vi "AeroQuadConfigurator.vi"() -> ()   [LabVIEW 2009]
uses:
  <vilib>/Utility/config.llb/Config Data RefNum.ctl
  <vilib>/Utility/config.llb/Read Key (Double).vi
  <vilib>/Utility/config.llb/Read Key (String).vi
  <vilib>/Utility/config.llb/Write Key (String).vi
  <vilib>/Utility/config.llb/Write Key (U32).vi
  <vilib>/Instr/_visa.llb/VISA Configure Serial Port (Instr).vi
  Instance           2 29Saved   MikroQuadConfigurator .vi
  <vilib>/Utility/error.llb/DialogType.ctl
  <vilib>/Utility/config.llb/NI_LVConfig.lvlib
  <vilib>/ptbypt/NI_PtbyPt.lvlib
panel:
  in  "ConfigGUI":T1(tab)
  in  "Communication Port":refnum<visa-resource-name>
  in  "Timeout (sec)":u32=4
  in  "Connect":bool
  in  "Disconnect":bool
  in  "UpdateAcro":bool
  in  "ProportionalPitch":dbl caption="Proportional" format="%.2f"
  in  "IntegralPitch":dbl caption="Integral" format="%.2f"
  in  "DerivativePitch":dbl caption="Derivative" format="%.2f"
  in  "Proportional Roll":dbl caption="Proportional" format="%.2f"
  in  "Integral Roll":dbl caption="Integral" format="%.2f"
  in  "Derivative Roll":dbl caption="Derivative" format="%.2f"
  in  "Windup Guard":dbl format="%.2f"
  in  "UpdateStable":bool
  in  "ProportionalRollLevel":dbl caption="Proportional" format="%.2f"
  in  "IntegralRollLevel":dbl caption="Integral" format="%.2f"
  in  "DerivativeRollLevel":dbl caption="Derivative" format="%.2f"
  in  "ProportionalPitchLevel":dbl caption="Proportional" format="%.2f"
  in  "IntegralPitchLevel":dbl caption="Integral" format="%.2f"
  in  "DerivativePitchLevel":dbl caption="Derivative" format="%.2f"
  in  "Level Limit":u16
  in  "Level Off":u16=1 min=1 step=1
  in  "ProportionalHeading":dbl caption="Proportional" format="%.2f"
  in  "IntegralHeading":dbl caption="Integral" format="%.2f"
  in  "DerivativeHeading":dbl caption="Derivative" format="%.2f"
  in  "ProportionalYaw":dbl caption="Proportional" format="%.2f"
  in  "IntegralYaw":dbl caption="Integral" format="%.2f"
  in  "DerivativeYaw":dbl caption="Derivative" format="%.2f"
  in  "UpdateYaw":bool
  in  "Gyro Smooth Factor":dbl=0.01 min=0.01 max=1.0 step=0.01 format="%.2f"
  in  "Acc Smooth Factor":dbl=0.01 min=0.01 max=1.0 step=0.01 format="%.2f"
  in  "Complementary Filter":dbl format="%.2f"
  in  "UpdateSensors":bool
  in  "CalibrateGyros":bool
  in  "CalibrateAccels":bool
  in  "Throttle Smoothing":dbl=0.01 min=0.01 max=1.0 step=0.01 format="%.2f"
  in  "Mode  Smoothing":dbl=0.01 min=0.01 max=1.0 step=0.01 format="%.2f"
  in  "Aux  Smoothing":dbl=0.01 min=0.01 max=1.0 step=0.01 format="%.2f"
  in  "Roll Smoothing":dbl=0.01 min=0.01 max=1.0 step=0.01 format="%.2f"
  in  "Pitch Smoothing":dbl=0.01 min=0.01 max=1.0 step=0.01 format="%.2f"
  in  "Yaw  Smoothing":dbl=0.01 min=0.01 max=1.0 step=0.01 format="%.2f"
  in  "UpdateXmit":bool
  in  "Transmitter Factor":dbl=0.01 min=0.01 max=1.0 step=0.01 format="%.2f"
  in  "CalibrateTransmitter":bool
  in  "DefaultTransmitterValue":bool
  in  "Transmitter Instructions 2":string="Before starting the transmitter calibration, set the transmitter to it's default settings.\n\nIt can be in Airplane or Helicopter mode.\n\nVerify that:\n- ESC's and motors are\n  disconnected from power! \n- Trims and subtrims are zero\n- End Point Adjustment (EPA) \n  are 100%"
  in  "Test Comments":string
  in  "SaveFlightData":bool
  in  "ViewFlightData":bool
  in  "InitializeEEPROM":bool
  in  "CalibrateTransmitterFront":bool
  in  "CalibrateESCs":bool
  in  "Minimum Test Throttle":dbl=1050.0 min=1000.0 max=1200.0
  in  "EEPROM Instructions":string="The first step to setting up your AeroQuad is to initialize the user configurable EEPROM with default values. \n\nSelect the \"Initialize EEPROM\" button to set the EEPROM to default values."
  in  "Transmitter Instructions":string="The next step is to calibrate your transmitter. Before starting the calibration, set the\ntransmitter to it's default settings.\n\nIt can be in Airplane or Helicopter mode.\n\nVerify that:\n- ESC's and motors are\n  disconnected from power! \n- Trims and subtrims are zero\n- End Point Adjustment (EPA) \n  are 100%"
  in  "ESC Instructions":string="Before your first flight, perform an ESC throttle calibration per the manufacturer's instructions.  This cal procedure is implemented specifically for the Turnigy line of ESC's.\n\nThe flight control board will need to be powered separately from the ESC's motors.  Use the USB cable to power the flight control board, and a battery to power the ESC's/motors.\n\nInsure that there is no power applied to the ESC's and motors before the start of calibration."
  in  "PerformPreFlightCheckout":bool
  in  "GUI":T2(tab)
  out "Yaw":i16(knob) scale=-200.0..200.0
  out "Pitch":i16(knob) scale=-200.0..200.0
  out "Rear Motor":i16(slide) scale=1000.0..2000.0
  out "Front Motor":i16(slide) scale=1000.0..2000.0
  out "Left Motor":i16(slide) scale=1000.0..2000.0
  out "Right Motor":i16(slide) scale=1000.0..2000.0
  out "Motor Commands":T3(graph)
  in  "Motor Plot":enum16{"Motor Chart", "Motor Bar Plot"}(ring)
  in  "Output Type":T4(ring)
  out "Roll":i16(knob) scale=-200.0..200.0
  out "PID / Sensor Output":cluster{"[0]":i16, "[1]":i16, "[2]":i16}(graph)
  out "Mode 2":bool caption="Flight Mode"
  out "Armed":bool caption="Motor Output Status"
  out "Loop Rate":i16
  out "Pitch Angle":dbl(knob) scale=-180.0..180.0
  out "Roll Angle":dbl(knob) scale=-180.0..180.0
  in  "Plot 10":bool=TRUE
  in  "Plot 9":bool=TRUE
  in  "Plot 8":bool=TRUE
  in  "Plot 7":bool=TRUE
  in  "Plot 6":bool=TRUE
  in  "Plot 5":bool=TRUE
  in  "Plot 4":bool=TRUE
  in  "Plot 3":bool=TRUE
  in  "Plot 2":bool=TRUE
  in  "Plot 1":bool=TRUE
  out "Auto Level Pitch":cluster{i16, i16}(slide) scale=-50.0..50.0
  out "Auto Level Roll":cluster{i16, i16}(slide) scale=-50.0..50.0
  out "Raw Data":T5(graph)
  out "Aux":cluster{i16, i16, i16}(slide)={2000, 1000, 1000} scale=1000.0..2000.0
  out "Mode":cluster{i16, i16, i16}(slide)={2000, 1000, 1000} scale=1000.0..2000.0
  out "Roll Channel":cluster{i16, i16, i16}(slide)={2000, 1000, 1500} scale=1000.0..2000.0
  out "Pitch Channel":cluster{i16, i16, i16}(slide)={2000, 1000, 1500} scale=1000.0..2000.0
  out "Yaw Channel":cluster{i16, i16, i16}(slide)={2000, 1000, 1500} scale=1000.0..2000.0
  out "Throttle Channel":cluster{i16, i16, i16}(slide)={2000, 1000, 1000} scale=1000.0..2000.0
  out "Transmitter Factor Indicator":dbl caption="Transmitter Factor" format="%.2f"
  in  "Plot 18":bool=TRUE
  in  "Plot 17":bool=TRUE
  in  "Plot 16":bool=TRUE
  in  "Plot 15":bool=TRUE
  in  "Plot 14":bool=TRUE
  in  "Plot 13":bool=TRUE
  in  "Plot 12":bool=TRUE
  in  "Plot 11":bool=TRUE
  out "Command Data":T6(graph)
  in  "MotorScale":u16(ring) caption="Motor Scale Display" items=["Low Scale", "Full Scale"]
  in  "KillMotorCommand":bool
  in  "SendMotorCommand":bool
  in  "LeftMotorCommand":i32(slide)=1000 caption="Left" min=1000 max=2000 step=1 scale=1000.0..1200.0
  in  "Right MotorCommand":i32(slide)=1000 caption="Right" min=1000 max=2000 step=1 scale=1000.0..1200.0
  in  "RearMotorCommand":i32(slide)=1000 caption="Rear" min=1000 max=2000 step=1 scale=1000.0..1200.0
  in  "FrontMotorCommand":i32(slide)=1000 caption="Front" min=1000 max=2000 step=1 scale=1000.0..1200.0
  out "Transmitter Yaw Command":dbl(slide)=1500.0 scale=1000.0..2000.0
  out "DeltaHeading":dbl(graph)
  out "Delta Heading":dbl
  out "Heading":cluster{dbl, dbl}(knob)={0.0, 90.0} scale=-180.0..180.0
  in  "NoneFound":string="No Frequencies Detected"
  out "Bytes To Process":u32(slide) scale=0.0..64000.0 scale format="%.0p"
  in  "ResetFFT":bool
  out "Time Domain":i16(graph)
  out "Max Frequency Detected":dbl format="%.1f"
  in  "Signal":i32(ring) items=["Roll Gyro", "Pitch Gyro", "Yaw Gyro", "Roll Acc", "Pitch Acc"]
  out "Frequency Domain":T7(graph)
  out "SerialData":string
  in  "Command":string
  in  "SendCommand":bool
  in  "UserConfigSelect":u16(ring) items=["Connect", "Acrobatic Mode", "Stable Mode", "Yaw Configuration", "Sensors", "Transmitter", "Data Storage", "Initial Setup"]
  in  "PlotSelection":u16(ring) items=["Flight Configuration", "Raw Sensor Data", "Transmitter Adjustment", "Transmitter Data", "Motor Commands", "Heading Hold", "Spectrum Analyzer", "Serial Monitor"]
  out "Flight Software Version":string
  out "Status":string
  # "To arm the motor output\nmove the throttle transmitter\nstick to the lower right.\n\nTo disarm the motor output\nmove the throttle transmitter\nstick to the lower left."
  # "Roll  PID Values"
  # "Pitch PID Values"
  # "Roll Level PID Values"
  # "Pitch Level PID Values"
  # "Note:  This is an experimental\nfeature and is still under\ndevelopment.  By default it is\ndisabled in the flight control\nsoftware.  To enable, remove\nthe comment before the\nappropriate #define\nstatement in AeroQuad.pde."
  # "Yaw PID Values"
  # "Heading Hold  PID Values"
  # "A sensor calibration for both\ngyros and acceleromters\ncan be performed manually\nfrom the transmitter.\n\nMove the left transmitter stick\nto the lower left hand corner\nand the right stick to the lower\nright hand corner.\n\nThe motors will pulse three\ntimes to confirm the calibration\nis completed."
  # "All sensor data is automatically\nstored in C:\\TestData."
  # "Roll Level"
  # "Pitch Level"
  # "Roll Adjust"
  # "Pitch Adjust"
  # "Max"
  # "Max"
  # "Max"
  # "Min"
  # "Min"
  # "Max"
  # "Max"
  # "Max"
  # "Min"
  # "Min"
  # "Min"
  # "Min"
  # "Warning!  It is strongly recommended\nto remove the propellers from the\nmotors before sending motor\ncommands from the Configurator."
  # "Note:  By default heading hold is\ndisabled in the flight control\nsoftware. To enable, remove\nthe comment before the\nappropriate #define\nstatement in AeroQuad.pde."
  # "If you experience a continuous yaw\nin one direction, perform a sensor\ncalibration to update the gyro cal."
  # "1475"
  # "1525"
  # "Heading Hold Off"
  # "On"
  # "Heading Hold Off"
  # "Commanded Heading"
  # "Hz"
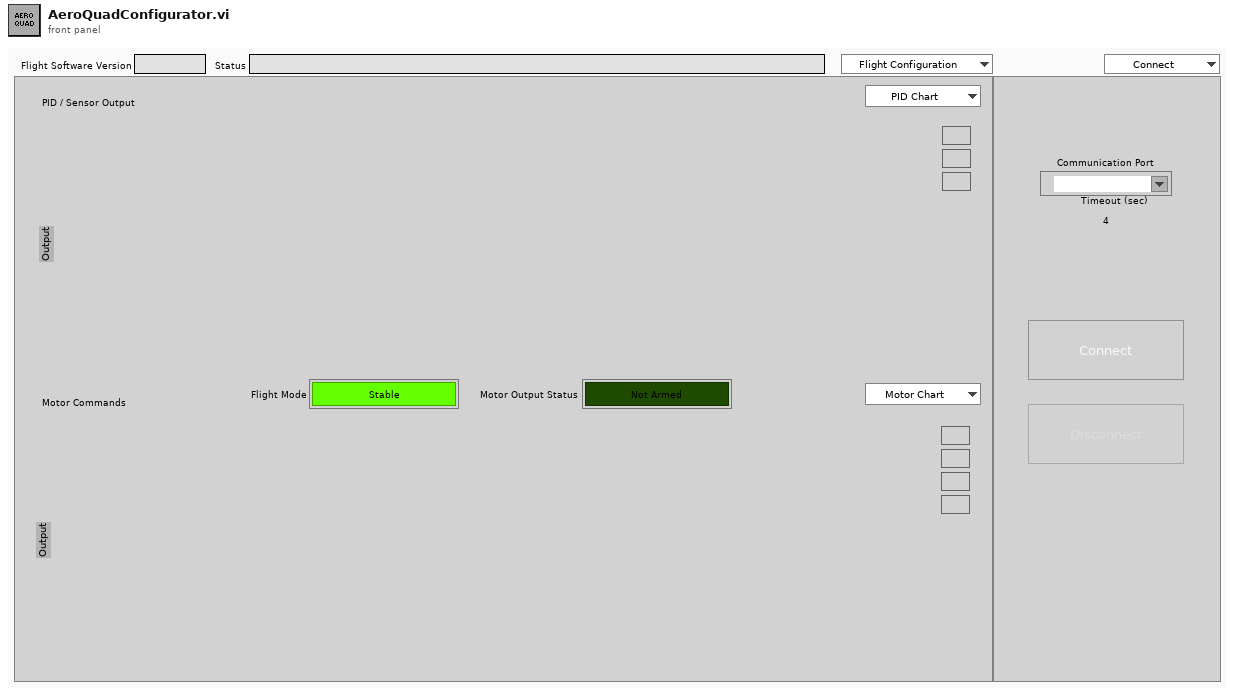
[diagram p1: front panel]
types:
  T1 = enum32{"Connect", "Acrobatic Mode", "Stable Mode", "Yaw Configuration", "Sensors", "Transmitter", "Data Storage", "Initial Setup", "Pre-Flight Checkout"}
  T2 = enum32{"Flight Configuration", "Raw Sensor Data", "Transmitter Adjustment", "Transmitter Data", "Motor Commands", "Heading Hold", "Spectrum Analyzer", "Serial Monitor"}
  T3 = cluster{"[0]":i16, "[1]":i16, "[2]":i16, "[3]":i16}
  T4 = enum16{"PID Chart", "Gyro Chart", "Gyro Indicators"}
  T5 = cluster{"[0]":dbl, "[1]":dbl, "[2]":dbl, "[3]":dbl, "[4]":dbl, "[5]":dbl, "[6]":dbl, "[7]":dbl, "[8]":dbl, "[9]":dbl}
  T6 = cluster{"[0]":i16, "[1]":i16, "[2]":i16, "[3]":i16, "[4]":i16, "[5]":i16, "[6]":i16, "[7]":i16}
  T7 = cluster{dbl, "df":dbl, "Power Spectrum (V^2 rms)":dbl[]}
  T8 = enum8{"Enabled", "Disabled", "Disabled and Grayed Out"}
  T9 = cluster{"[0]":i16, "[1]":i16, "[2]":i16, "[3]":i16}[]
  T10 = typedef "NI_LVConfig.lvlib/Config Data RefNum.ctl" = refnum<k1>
  T11 = cluster{"Error":errorcluster, "Debug":bool, "COMport":refnum<visa-resource-name>, "Connected":bool, "CheckConfig":string, "WorkingPath":path, "INIref":T10, "ConnectType":bool, "360/PI":dbl, "Save":bool, "DataRef":refnum<k34>, "CurrentTime":timestamp, "dT":dbl, "MinLimits":i16[], "MaxLimits":i16[], "Retry":i32, "CurrentRetry":i32, "FlightVersion":dbl, "Output Type":enum16{"PID Chart", "Gyro Chart", "Gyro Indicators"}, "Motor Plot":enum16{"Motor Chart", "Motor Bar Plot"}, "Timeout":u32, "ResetFFT":bool, "AREF":dbl}
  T12 = enum16{"open", "open or create", "create or replace", "create", "open (read-only)"}
  T13 = enum32{"invalid app kind", "Development System", "Run Time System", "Student Edition", "Embedded LabVIEW", "Evaluation", "Custom"}
  T14 = typedef "DialogType.ctl" = u16
  T15 = cluster{"[0]":i16, "[1]":i16, "[2]":i16, "[3]":i16, "[4]":i16, "[5]":i16, "[6]":i16, "[7]":i16}[]
  T16 = cluster{"[0]":dbl, "[1]":dbl, "[2]":dbl, "[3]":dbl, "[4]":dbl, "[5]":dbl, "[6]":dbl, "[7]":dbl, "[8]":dbl, "[9]":dbl}[]
  T17 = typedef "eventvkey.ctl" = enum16{"ASCII", "Enter", "Return", "Shift", "Ctrl", "Alt", "Cmd", "Opt", "Caps", "NumLock", "Clear", "Break", "Up", "Down", "Left", "Right", "Insert", "Delete", "Home", "End", "PageUp", "PageDown", "Escape", "Help", "Pause", "ScrollLock", "F1", "F2", "F3", "F4", "F5", "F6", "F7", "F8", "F9", "F10", "F11", "F12", "F13", "F14", "F15", "F16", "F17", "F18", "F19", "F20", "F21", "F22", "F23", "F24", "Play", "VolumeUp", "VolumeDown", "Mute", "Two Byte Char"}
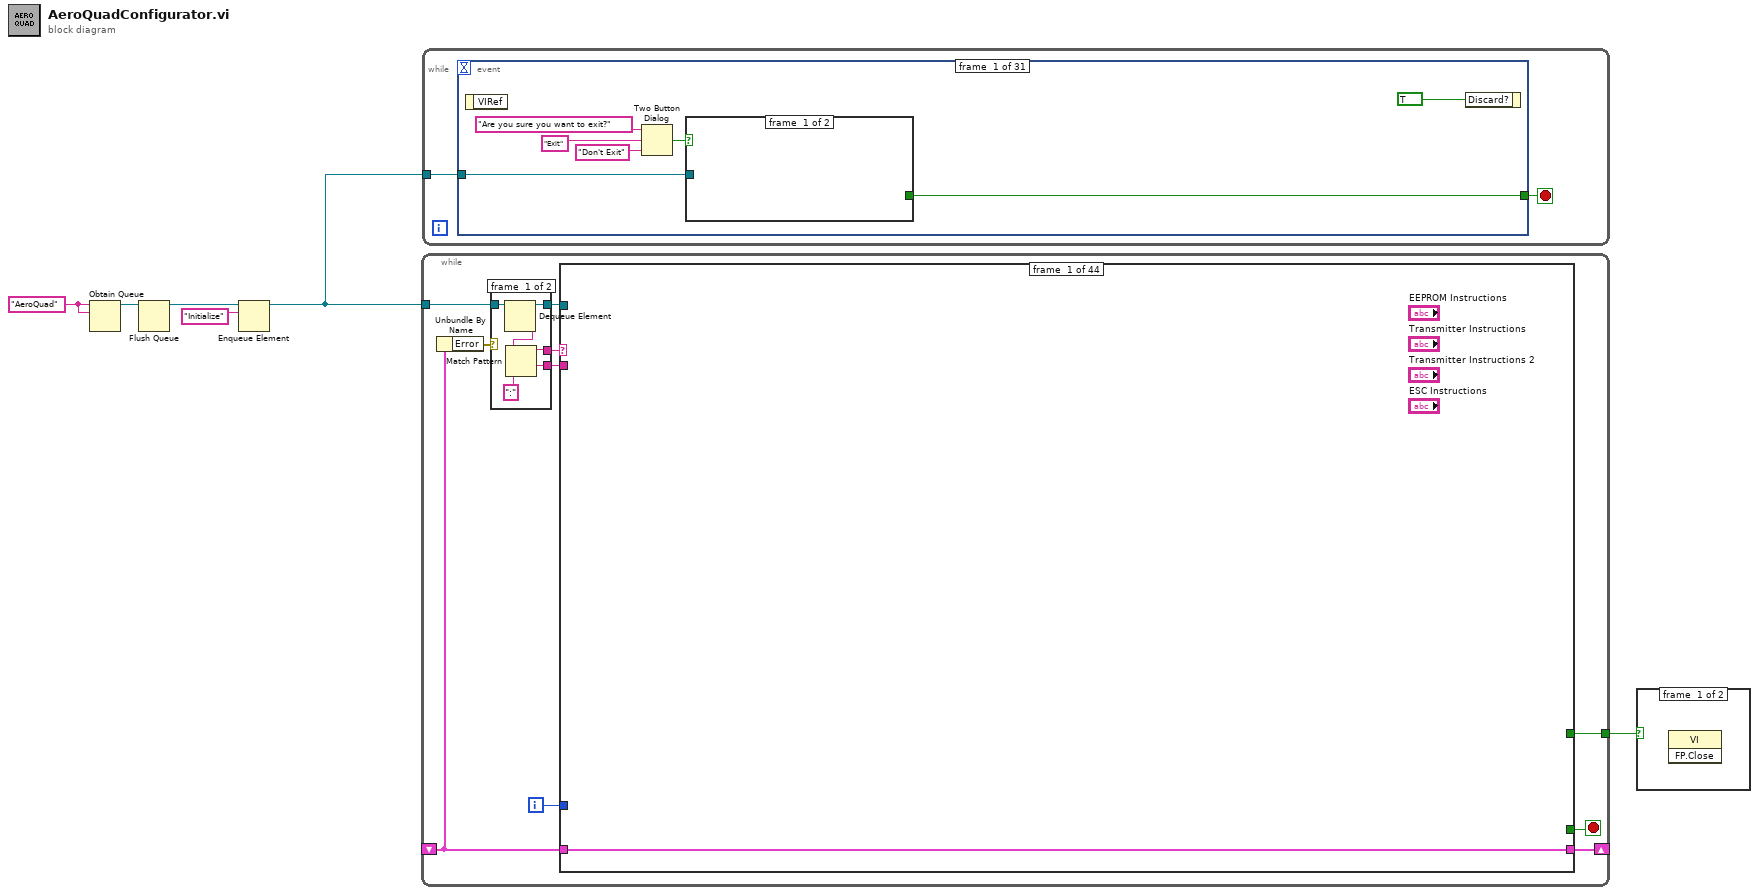
[diagram p0: block diagram]
diagram:
  w5 = "AeroQuad" ("name (unnamed)")
  n1 = Obtain Queue(name (unnamed)=w5, element data type=w5) -> (queue out=w3:refnum<queue>)  [unwired: 3 in, 2 out]
  n2 = Flush Queue(queue=w3) -> (queue out=w2:refnum<queue>)  [unwired: 1 in, 2 out]
  n3 = Enqueue Element(queue=w2, element="Initialize") -> (queue out=w4:refnum<queue>)  [unwired: 1 in, 3 out]
  n4 = while {
    shift-right: [w16] -> _
    shift-left: _ -> [w11]
    tunnel: w4 -> [w13]
    tunnel: [w8] -> w1
    i -> [w9]
    stop <- w15 stop-if-true
    n5 = Unbundle By Name(w11) -> ("Error"=w10:errorcluster)
    n6 = case shown="No Error" w10 {
      tunnel: [w20 "Error" ("name (unnamed)")] -> w14
      tunnel: w13 -> [w22 w24]
      tunnel: [w21 w24] -> w12
      tunnel: [w19 _] -> w7
      frame #0 {
        n7 = Dequeue Element(queue=w22) -> (queue out=w21:refnum<queue>, element=w18:string)  [unwired: 1 in, 3 out]
        n8 = Match Pattern(string=w18, regular expression=":") -> (before substring=w20:string, after substring=w19:string)  [unwired: 3 out]
      }
      frame #1 {
      }
    }
    n9 = case shown="\"Calibrate ESC's\"" w14 {
      tunnel: w12 -> [_ w55 _ _ w116 _ _ _ _ _ _ _ w192 _ w198 w237 w277 _ w375 w401 w427 w455 w467 _ w486 w489 _ _ _ w671 w706 w759 w770 w803 w816 w843 _ _ _ _ _ _ _ _]
      selector: w14 -> [_ _ _ _ _ _ _ _ _ _ _ w187 _ _ _ _ _ _ _ _ _ _ _ _ _ _ _ _ _ _ _ _ _ _ _ _ _ _ _ _ _ _ _ w1101]
      tunnel: [w25 w56 w78 w85 w120 w139 w148 w168 w177 w181 w183 w185 w195 w197 w210 w241 w256 w305 w377 w403 w429 w464 w470 w475 w487 w498 w564 w635 w637 w676 w712 w748 w772 w804 w825 w841 w886 w892 w934 w963 w1012 w1059 w1089 w1098] -> w16
      tunnel: w11 -> [w25 _ w79 w85 w121 w139 w149 w169 w177 w181 w184 w185 w195 w197 w213 w238 w262 w304 w378 w405 w431 w465 w470 w475 w488 w499 w565 w636 w637 w677 w713 w749 w773 w805 w826 w839 w886 w893 w936 w965 w1013 w1060 w1089 w1096]
      tunnel: [_ _ _ _ _ _ _ _ _ _ _ _ TRUE _ _ _ _ _ _ _ _ _ _ _ _ _ _ _ _ _ _ _ _ _ _ _ _ _ _ _ _ _ _ _] -> w15
      tunnel: w9 -> [_ _ _ _ w119 _ _ _ _ _ _ _ _ _ _ _ _ _ _ _ _ _ _ _ _ _ _ _ _ _ _ _ _ _ _ _ _ _ _ _ _ _ _ _]
      tunnel: [_ _ _ _ _ _ _ _ _ _ _ _ w193 _ _ _ _ _ _ _ _ _ _ _ _ _ _ _ _ _ _ _ _ _ _ _ _ _ _ _ _ _ _ _] -> w8
      tunnel: w7 -> [_ _ _ _ _ _ _ _ w176 w180 _ _ _ _ _ _ _ _ _ w400 w426 _ _ _ _ _ _ _ _ _ _ _ _ _ _ _ _ _ _ _ _ _ _ _]
      frame #0 {
      }
      frame #1 {
        w32 = 0
        w30 = T8."Disabled and Grayed Out" ("Disabled")
        w36 = FALSE ("Visible")
        w38 = FALSE ("Visible")
        n10 = Enqueue Element(queue=w55, element="Load Config") -> (queue out=w50:refnum<queue>)  [unwired: 1 in, 3 out]
        n11 = local write "Motor Plot"(enum16{"Motor Chart", "Motor Bar Plot"}."Motor Chart" ("Motor Plot")) -> ()
        n12 = local write "Output Type"(T4."PID Chart" ("Output Type")) -> ()
        n13 = Enqueue Element(queue=w50, element="Modify Plots") -> (queue out=w45:refnum<queue>)  [unwired: 1 in, 3 out]
        n14 = property on="Connect" class="Bool"("Disabled"=T8."Enabled") -> ()  [unwired: 2 in, 2 out]
        n15 = property on="PID / Sensor Output" class="WFChart (strict)"("Visible"=TRUE) -> ()  [unwired: 2 in, 2 out]
        n16 = Current VI's Path() -> (path=w52:path)
        n17 = property class="App"() -> ("App.Kind"=w58:T13)  [unwired: 2 in, 2 out]
        n18 = Strip Path(path=w52) -> (stripped path=w53:path)  [unwired: 1 out]
        n19 = Enqueue Element(queue=w45, element="Status: Not Connected to AeroQuad") -> ()  [unwired: 1 in, 4 out]
        n20 = local write "GUI"(w32) -> ()
        n21 = local write "ConfigGUI"(w32) -> ()
        n22 = local write "PlotSelection"(w32) -> ()
        n23 = local write "UserConfigSelect"(w32) -> ()
        n24 = case shown="\"Development System\"" w58 {
          tunnel: w53 -> [w59 w61]
          tunnel: [w59 w60] -> w47
          frame #0 {
          }
          frame #1 {
            n25 = Strip Path(path=w61) -> (stripped path=w60:path)  [unwired: 1 out]
          }
        }
        n26 = property on="Motor Commands" class="WFChart (strict)"("History Data"=T9 [], "Visible"=TRUE) -> ()  [unwired: 2 in, 2 out]
        n27 = property on="DefaultTransmitterValue" class="Bool"("Disabled"=u8 2) -> ()  [unwired: 2 in, 2 out]
        n28 = property on="PID / Sensor Output" class="WFChart (strict)"("History Data"=cluster{"[0]":i16, "[1]":i16, "[2]":i16}[] [], "YScale.Maximum"=1200.0 ("Y Scale.Range:Maximum"), "YScale.Minimum"=-1200.0 ("Y Scale.Range:Minimum")) -> ()  [unwired: 2 in, 2 out]
        n29 = property on="PerformPreFlightCheckout" class="Bool"("Disabled"=w30) -> ()  [unwired: 2 in, 2 out]
        n30 = property on="InitializeEEPROM" class="Bool"("Disabled"=w30) -> ()  [unwired: 2 in, 2 out]
        n31 = property on="SaveFlightData" class="Bool (strict)"("DisabledEnum"=w30) -> ()  [unwired: 2 in, 2 out]
        n32 = property on="UpdateAcro" class="Bool"("DisabledEnum"=w30) -> ()  [unwired: 2 in, 2 out]
        n33 = property on="UpdateSensors" class="Bool"("DisabledEnum"=w30) -> ()  [unwired: 2 in, 2 out]
        n34 = property on="UpdateStable" class="Bool"("DisabledEnum"=w30) -> ()  [unwired: 2 in, 2 out]
        n35 = property on="UpdateXmit" class="Bool"("DisabledEnum"=w30) -> ()  [unwired: 2 in, 2 out]
        n36 = Divide(x=-360.0, y=3.141592653589793) -> (x/y=w29:dbl)
        n37 = Divide(x=2.892 ("AREF"), y=1024.0 ("AREF")) -> (x/y=w26:dbl)
        n38 = property on="Roll" class="Knob (strict)"("Visible"=w38) -> ()  [unwired: 2 in, 2 out]
        n39 = property on="Pitch" class="Knob (strict)"("Visible"=w38) -> ()  [unwired: 2 in, 2 out]
        n40 = property on="Yaw" class="Knob (strict)"("Visible"=w38) -> ()  [unwired: 2 in, 2 out]
        n41 = Bundle By Name(cluster=T11 {"Error"={"status"=FALSE, "code"=0, "source"=""}, "Debug"=FALSE, "COMport"="", "Connected"=FALSE, "CheckConfig"="", "WorkingPath"=path "", "INIref"=refnum, "ConnectType"=FALSE, "360/PI"=0.0, "Save"=FALSE, "DataRef"=refnum, "CurrentTime"=timestamp(0 s since 1904-01-01), "dT"=0.0, "MinLimits"=[1000, 1000, 1000, 1000, 1000, 1000], "MaxLimits"=[2000, 2000, 2000, 2000, 2000, 2000], "Retry"=0, "CurrentRetry"=0, "FlightVersion"=1.4, "Output Type"=enum."PID Chart", "Motor Plot"=enum."Motor Chart", "Timeout"=0, "ResetFFT"=TRUE, "AREF"=0.0}, "WorkingPath"=w47, "360/PI"=w29, "AREF"=w26) -> (w56:T11)
        n42 = property on="SendMotorCommand" class="Bool"("DisabledEnum"=w30) -> (error out=w31:errorcluster)  [unwired: 2 in, 1 out]
        n43 = property on="Disconnect" class="Bool"("Disabled"=w30) -> ()  [unwired: 2 in, 2 out]
        n44 = property on="CalibrateESCs" class="Bool"("Disabled"=w30) -> ()  [unwired: 2 in, 2 out]
        n45 = property on="CalibrateTransmitterFront" class="Bool"("Disabled"=w30) -> ()  [unwired: 2 in, 2 out]
        n46 = property on="CalibrateTransmitter" class="Bool"("Disabled"=w30) -> ()  [unwired: 2 in, 2 out]
        n47 = property on="UpdateXmit" class="Bool"("DisabledEnum"=w30) -> ()  [unwired: 2 in, 2 out]
        n48 = property on="SendCommand" class="Bool"("DisabledEnum"=w30) -> ()  [unwired: 2 in, 2 out]
        n49 = property on="CalibrateGyros" class="Bool"("DisabledEnum"=w30) -> ()  [unwired: 2 in, 2 out]
        n50 = property on="CalibrateAccels" class="Bool"(error in=w31, "DisabledEnum"=w30) -> ()  [unwired: 1 in, 2 out]
        n51 = property on="Front Motor" class="Slide (strict)"("Visible"=w36) -> ()  [unwired: 2 in, 2 out]
        n52 = property on="Rear Motor" class="Slide (strict)"("Visible"=w36) -> ()  [unwired: 2 in, 2 out]
        n53 = property on="Right Motor" class="Slide (strict)"("Visible"=w36) -> ()  [unwired: 2 in, 2 out]
        n54 = property on="Left Motor" class="Slide (strict)"("Visible"=w36) -> ()  [unwired: 2 in, 2 out]
      }
      frame #2 {
        w74 = "Configuration" ("section")
        n55 = Unbundle By Name(w79) -> ("WorkingPath"=w72:path, "Error"=w70:errorcluster)
        n56 = Build Path(base path=w72, name or relative path="AeroQuadConfigurator.ini") -> (appended path=w71:path)
        n57 = call <vilib>:"Open Config Data (compatibility).vi"("error in (no error)"=w70, "configuration file path"=w71) -> ("error out"=w68:errorcluster, "refnum"=w69:T10)  [unwired: 7 in, 1 out]
        n58 = call <vilib>:"Get Section Names.vi"("error in (no error)"=w68, "refnum"=w69) -> ("error out"=w67:errorcluster, "refnum out"=w66:T10)  [unwired: 8 out]
        n59 = call-poly <vilib>:"Read Key.vi"("section"=w74, "error in (no error)"=w67, "default value"="COM2", "key"="COMport", "refnum"=w66) -> ("error out"=w62:errorcluster, "value"=w80:string, "refnum out"=w65:T10)  [unwired: 1 in, 3 out]
        n60 = property on="Communication Port" class="VISAName"("Value"=w80) -> ()  [unwired: 2 in, 2 out]
        n61 = call-poly <vilib>:"Read Key.vi"("section"=w74, "error in (no error)"=w62, "default value"=5.0, "key"="Timeout", "refnum"=w65) -> ("error out"=w63:errorcluster, "value"=w76:dbl, "refnum out"=w64:T10)  [unwired: 4 out]
        n62 = local write "Timeout (sec)"(w76) -> ()
        n63 = Bundle By Name(cluster=w79, "INIref"=w64, "Error"=w63) -> (w78:T11)
      }
      frame #3 {
        n64 = Build Array("Plot 1", "Plot 2", "Plot 3", "Plot 4", "Plot 5", "Plot 6", "Plot 7", "Plot 8", "Plot 9", "Plot 10") -> (w95:bool[])
        n65 = Build Array("Plot 11", "Plot 12", "Plot 13", "Plot 14", "Plot 15", "Plot 16", "Plot 17", "Plot 18") -> (w86:bool[])
        n66 = for {
          tunnel: w86 -> [w105] mode=indexing
          i -> [w104]
          n67 = property on="Command Data" class="WFChart (strict)"("Active Plot"=w104, "Plot.Visible?"=w105) -> ()  [unwired: 2 in, 2 out]
        }
        n68 = for {
          tunnel: w95 -> [w107] mode=indexing
          i -> [w106]
          n69 = property on="Raw Data" class="WFChart (strict)"("Active Plot"=w106, "Plot.Visible?"=w107) -> ()  [unwired: 2 in, 2 out]
        }
      }
      frame #4 {
        w108 = u8 0 ("Disabled")
        n70 = Flush Queue(queue=w116) -> (queue out=w115:refnum<queue>)  [unwired: 1 in, 2 out]
        n71 = Unbundle By Name(w121) -> ("Connected"=w110:bool, "Error"=w123:errorcluster, "COMport"=w111:refnum<visa-resource-name>)
        n72 = VISA Flush I/O Buffer(VISA resource name=w111) -> (VISA resource name out=w113:refnum<visa-resource-name>, error out=w112:errorcluster)  [unwired: 1 in, 1 out]
        n73 = Enqueue Element(queue=w115, element="Initialize") -> (queue out=w109:refnum<queue>)  [unwired: 1 in, 3 out]
        n74 = VISA Close(VISA resource name=w113, error in (no error)=w112) -> ()  [unwired: 1 out]
        n75 = case shown="True" w110 {
          tunnel: w123 -> [w126 w136]
          tunnel: [w125 w137] -> w122
          tunnel: w119 -> [w124 _]
          tunnel: w109 -> [_ w132]
          frame #0 {
            n76 = case shown="Default" w124 {
              tunnel: w126 -> [w128 w129]
              tunnel: [w127 w131] -> w125
              frame #0 {
                n77 = call <vilib>:"Clear Errors.vi"("error in (no error)"=w128) -> ("error out"=w127:errorcluster)  [unwired: 6 out]
              }
              frame #1 {
                n78 = call "ErrorDialog.vi"("error in"=w129) -> ("error out"=w130:errorcluster)  [unwired: 10 out]
                n79 = call <vilib>:"Clear Errors.vi"("error in (no error)"=w130) -> ("error out"=w131:errorcluster)  [unwired: 6 out]
              }
            }
          }
          frame #1 {
            n80 = Enqueue Element(queue=w132, element="Status:Not Connected to AeroQuad") -> (queue out=w134:refnum<queue>)  [unwired: 1 in, 3 out]
            n81 = call <vilib>:"Clear Errors.vi"("error in (no error)"=w136) -> ("error out"=w137:errorcluster)  [unwired: 6 out]
            n82 = Enqueue Element(queue=w134, element="Connection Retry Dialog") -> ()  [unwired: 1 in, 4 out]
          }
        }
        n83 = Bundle By Name(cluster=w121, "Connected"=FALSE, "Error"=w122) -> (w120:T11)
        n84 = property on="Connect" class="Bool"("Disabled"=w108) -> ()  [unwired: 2 in, 2 out]
        n85 = local write "GUI"(w108) -> ()
        n86 = local write "ConfigGUI"(w108) -> ()
        n87 = local write "Status"("Lost connection to AeroQuad" ("Connection Status")) -> ()
      }
      frame #5 {
        n88 = One Button Dialog(message="AeroQuad Configurator v1.3.2") -> ()  [unwired: 2 out]
      }
      frame #6 {
        n89 = Bundle By Name(cluster=w149, "Output Type"="Output Type") -> (w148:T11)
        n90 = case shown="\"Gyro Indicators\"" "Output Type" {
          tunnel: [300.0 ("Y Scale.Range:Maximum") 1500.0 ("Y Scale.Range:Maximum") 300.0 ("Y Scale.Range:Maximum")] -> w146
          tunnel: [-300.0 ("Y Scale.Range:Minimum") -1500.0 ("Y Scale.Range:Minimum") -300.0 ("Y Scale.Range:Minimum")] -> w145
          tunnel: [cluster{"[0]":i16, "[1]":i16, "[2]":i16}[] [] ("History Data") cluster{"[0]":i16, "[1]":i16, "[2]":i16}[] [] ("History Data") _] -> w144
          tunnel: [TRUE TRUE _] -> w143
          tunnel: [_ _ w158] -> w142
          tunnel: [_ _ w158] -> w141
          tunnel: [_ _ w158] -> w140
          frame #0 {
          }
          frame #1 {
          }
          frame #2 {
            w158 = TRUE
          }
        }
        n91 = property on="PID / Sensor Output" class="WFChart (strict)"("Visible"=w143, "History Data"=w144, "YScale.Maximum"=w146, "YScale.Minimum"=w145) -> ()  [unwired: 2 in, 2 out]
        n92 = property on="Roll" class="Knob (strict)"("Visible"=w142) -> ()  [unwired: 2 in, 2 out]
        n93 = property on="Pitch" class="Knob (strict)"("Visible"=w141) -> ()  [unwired: 2 in, 2 out]
        n94 = property on="Yaw" class="Knob (strict)"("Visible"=w140) -> ()  [unwired: 2 in, 2 out]
      }
      frame #7 {
        n95 = case shown="\"Motor Chart\", Default" "Motor Plot" {
          tunnel: [T9 [] ("History Data") _] -> w162
          tunnel: [TRUE FALSE] -> w161
          tunnel: [w170 w173] -> w166
          tunnel: [w170 w173] -> w165
          tunnel: [w170 w173] -> w164
          tunnel: [w170 w173] -> w163
          frame #0 {
            w170 = FALSE
          }
          frame #1 {
            w173 = TRUE
          }
        }
        n96 = Bundle By Name(cluster=w169, "Motor Plot"="Motor Plot") -> (w168:T11)
        n97 = property on="Front Motor" class="Slide (strict)"("Visible"=w166) -> ()  [unwired: 2 in, 2 out]
        n98 = property on="Rear Motor" class="Slide (strict)"("Visible"=w165) -> ()  [unwired: 2 in, 2 out]
        n99 = property on="Right Motor" class="Slide (strict)"("Visible"=w164) -> ()  [unwired: 2 in, 2 out]
        n100 = property on="Left Motor" class="Slide (strict)"("Visible"=w163) -> ()  [unwired: 2 in, 2 out]
        n101 = property on="Motor Commands" class="WFChart (strict)"("History Data"=w162, "Visible"=w161) -> ()  [unwired: 2 in, 2 out]
      }
      frame #8 {
        n102 = call <vilib>:"Trim Whitespace.vi"("string"=w176) -> ("trimmed string"=→"Status":string)  [unwired: 1 in]
      }
      frame #9 {
        n103 = Match Pattern(string=w180, regular expression=",") -> (before substring=w178:string)  [unwired: 4 out]
        n104 = One Button Dialog(message=w178) -> ()  [unwired: 2 out]
      }
      frame #10 {
        n105 = Bundle By Name(cluster=w184, "ResetFFT"=TRUE) -> (w183:T11)
      }
      frame #11 {
        n106 = Format Into String(format string="Unknown state encountered:\n%s", w187) -> (resulting string=w186:string)  [unwired: 2 in, 1 out]
        n107 = One Button Dialog(message=w186) -> ()  [unwired: 2 out]
      }
      frame #12 {
        n108 = Unbundle By Name(w195) -> ("INIref"=w189:T10, "COMport"=w194:refnum<visa-resource-name>, "Debug"=w193:bool)
        n109 = VISA Close(VISA resource name=w194) -> ()  [unwired: 1 in, 1 out]
        n110 = call <vilib>:"Close Config Data.vi"("refnum"=w189) -> ()  [unwired: 2 in, 9 out]
        n111 = Enqueue Element(queue=w192, element="Status:Disconnected from AeroQuad") -> (queue out=w191:refnum<queue>)  [unwired: 1 in, 3 out]
        n112 = Release Queue(queue=w191) -> ()  [unwired: 1 in, 4 out]
      }
      frame #13 {
      }
      frame #14 {
        w205 = "Configuration" ("section")
        n113 = Enqueue Element(queue=w198, element="Status:Initialize COM Port") -> (queue out=w199:refnum<queue>)  [unwired: 1 in, 3 out]
        n114 = Unbundle By Name(w213) -> ("INIref"=w201:T10)
        n115 = local read "Timeout (sec)"() -> (w216:u32)
        n116 = Enqueue Element(queue=w199, element="Open COM Port") -> ()  [unwired: 1 in, 4 out]
        n117 = call-poly <vilib>:"Write Key.vi"("section"=w205, "value"=w216, "key"="Timeout", "refnum"=w201) -> ("error out"=w203:errorcluster, "refnum out"=w202:T10)  [unwired: 1 in, 5 out]
        n118 = local read "Communication Port"() -> (w204:refnum<visa-resource-name>)
        n119 = call-poly <vilib>:"Write Key.vi"("section"=w205, "error in (no error)"=w203, "value"=w204, "key"="COMport", "refnum"=w202) -> ("error out"=w208:errorcluster, "refnum out"=w207:T10)  [unwired: 1 in, 4 out]
        n120 = call <vilib>:"Close Config Data.vi"("error in (no error)"=w208, "refnum"=w207) -> ("error out"=w215:errorcluster, "file path"=w214:path)  [unwired: 1 in, 7 out]
        n121 = call <vilib>:"Open Config Data.vi"("error in (no error)"=w215, "configuration file path"=w214) -> ("error out"=w212:errorcluster, "refnum"=w211:T10)  [unwired: 7 in, 1 out]
        n122 = Bundle By Name(cluster=w213, "INIref"=w211, "Error"=w212) -> (w210:T11)
      }
      frame #15 {
        w229 = u16 0 items=["None", "XON/XOFF", "RTS/CTS", "XON/XOFF & RTS/CTS", "DTR/DSR", "XON/XOFF & DTR/DSR"] ("flow control (0:none)")
        w235 = i16 0 items=["Unknown"=-1, "Unasserted"=0, "Asserted"=1] ("Serial Settings:Modem Line Settings:Line DTR State")
        n123 = call-poly "VISA Configure Serial Port"("VISA resource name"="Communication Port", "timeout (10sec)"=u32 1000, "termination char\n(0xA = '\\n' = LF)"=u8 10 ("termination char\n(0xA = '\\n' = LF)"), "Enable Termination\nChar (T)"=TRUE ("Enable Termination\nChar (T)"), "baud rate (9600)"=u32 115200, "flow control (0:none)"=w229) -> ("VISA resource name out"=w231:refnum<visa-resource-name>, "error out"=w232:errorcluster)  [unwired: 3 in, 5 out]
        n124 = VISA Open(error in (no error)=w232, VISA resource name=w231) -> (VISA resource name=w225:refnum<visa-resource-name>, error out=w224:errorcluster)  [unwired: 3 out]
        n125 = VISA Set I/O Buffer Size(VISA resource name=w225, size (4096)=u32 64000, error in (no error)=w224) -> (VISA resource name out=w222:refnum<visa-resource-name>, error out=w223:errorcluster)  [unwired: 1 in]
        n126 = property class="Instr"(reference=w222, error in=w223, "DTR State"=w235) -> (reference out=w242:refnum<visa-resource-name>, error out=w236:errorcluster)
        n127 = Unbundle By Name(w236) -> ("status"=w240:bool)
        n128 = case shown="No Error" w236 {
          tunnel: w237 -> [w249 w251]
          frame #0 {
            w244 = 0
            w243 = T8."Enabled" ("Disabled")
            n129 = property on="UpdateAcro" class="Bool"("DisabledEnum"=w243) -> ()  [unwired: 2 in, 2 out]
            n130 = property on="UpdateSensors" class="Bool"("DisabledEnum"=w243) -> ()  [unwired: 2 in, 2 out]
            n131 = property on="UpdateStable" class="Bool"("DisabledEnum"=w243) -> ()  [unwired: 2 in, 2 out]
            n132 = property on="UpdateXmit" class="Bool"("DisabledEnum"=w243) -> ()  [unwired: 2 in, 2 out]
            n133 = property on="Disconnect" class="Bool"("Disabled"=w243) -> ()  [unwired: 2 in, 2 out]
            n134 = property on="PerformPreFlightCheckout" class="Bool"("Disabled"=w243) -> ()  [unwired: 2 in, 2 out]
            n135 = property on="InitializeEEPROM" class="Bool"("Disabled"=w243) -> ()  [unwired: 2 in, 2 out]
            n136 = property on="CalibrateTransmitterFront" class="Bool"("Disabled"=w243) -> ()  [unwired: 2 in, 2 out]
            n137 = property on="CalibrateTransmitter" class="Bool"("Disabled"=w243) -> ()  [unwired: 2 in, 2 out]
            n138 = property on="Connect" class="Bool"("Disabled"=T8."Disabled and Grayed Out") -> ()  [unwired: 2 in, 2 out]
            n139 = local write "GUI"(w244) -> ()
            n140 = local write "PlotSelection"(w244) -> ()
            n141 = Enqueue Element(queue=w249, element="Status:Connecting to AeroQuad") -> (queue out=w250:refnum<queue>)  [unwired: 1 in, 3 out]
            n142 = property on="DefaultTransmitterValue" class="Bool"("Disabled"=w243) -> ()  [unwired: 2 in, 2 out]
            n143 = property on="SaveFlightData" class="Bool (strict)"("DisabledEnum"=w243) -> ()  [unwired: 2 in, 2 out]
            n144 = property on="CalibrateESCs" class="Bool"("Disabled"=w243) -> ()  [unwired: 2 in, 2 out]
            n145 = property on="UpdateXmit" class="Bool"("DisabledEnum"=w243) -> ()  [unwired: 2 in, 2 out]
            n146 = property on="SendCommand" class="Bool"("DisabledEnum"=w243) -> ()  [unwired: 2 in, 2 out]
            n147 = local write "Flight Software Version"("" ("Flight Software Version")) -> ()
            n148 = property on="SendMotorCommand" class="Bool"("DisabledEnum"=w243) -> ()  [unwired: 2 in, 2 out]
            n149 = Enqueue Element(queue=w250, element="Connect to AeroQuad") -> ()  [unwired: 1 in, 4 out]
            n150 = property on="CalibrateGyros" class="Bool"("DisabledEnum"=w243) -> ()  [unwired: 2 in, 2 out]
            n151 = property on="CalibrateAccels" class="Bool"("DisabledEnum"=w243) -> ()  [unwired: 2 in, 2 out]
          }
          frame #1 {
            n152 = Enqueue Element(queue=w251, element="Disconnect") -> (queue out=w254:refnum<queue>)  [unwired: 1 in, 3 out]
            n153 = Enqueue Element(queue=w254, element="Connection Retry Dialog") -> ()  [unwired: 1 in, 4 out]
          }
        }
        n154 = Not(x=w240) -> (.not. x?=w239:bool)
        n155 = Compound Arithmetic op=MULTIPLY("Timeout (sec)", u32 1000 ("value")) -> (w219:u32)
        n156 = Bundle By Name(cluster=w238, "Connected"=w239, "COMport"=w242, "Error"=w236, "CurrentRetry"=0 ("Retry"), "Retry"="Timeout (sec)", "Timeout"=w219) -> (w241:T11)
      }
      frame #16 {
        n157 = Unbundle By Name(w262) -> ("CurrentRetry"=w263:i32, "Retry"=w264:i32, "FlightVersion"=w255:dbl, "COMport"=w272:refnum<visa-resource-name>)
        n158 = VISA Write(VISA resource name=w272, write buffer="X") -> (VISA resource name out=w273:refnum<visa-resource-name>, error out=w275:errorcluster)  [unwired: 1 in, 1 out]
        n159 = call "Time Delay4"("error in (no error)"=w275) -> ("error out"=w274:errorcluster)  [unwired: 1 in, 9 out]
        n160 = VISA Flush I/O Buffer(VISA resource name=w273, error in (no error)=w274) -> (VISA resource name out=w269:refnum<visa-resource-name>, error out=w271:errorcluster)  [unwired: 1 in]
        n161 = VISA Write(VISA resource name=w269, write buffer="!", error in (no error)=w271) -> (VISA resource name out=w267:refnum<visa-resource-name>, error out=w268:errorcluster)  [unwired: 1 out]
        n162 = VISA Read(VISA resource name=w267, byte count=u32 1024, error in (no error)=w268) -> (read buffer=w257:string, error out=w261:errorcluster)  [unwired: 2 out]
        n163 = Fract/Exp String To Number(string=w257) -> (number=w265:dbl)  [unwired: 4 out]
        n164 = Greater Or Equal?(x=w265, y=w255) -> (x >= y?=w258:bool)
        n165 = case shown="No Error" w261 {
          selector: w261 -> [w283 _]
          tunnel: [string[] ["Status:Connected to AeroQuad", "Read Configuration", "Configuration"] w294] -> w278
          tunnel: w264 -> [_ w298]
          tunnel: w263 -> [_ w292]
          tunnel: [w283 _] -> w260
          tunnel: [0 w297] -> w259
          tunnel: w258 -> [w281 _]
          tunnel: w257 -> [w282 _]
          tunnel: w255 -> [w279 _]
          frame #0 {
            n166 = case shown="False" w281 {
              tunnel: w279 -> [w287 _]
              frame #0 {
                n167 = Format Into String(format string="Flight Control Software version %.1f or higher\nis required to make all features of the Configurator to work properly." ("message"), w287) -> (resulting string=w285:string)  [unwired: 2 in, 1 out]
                n168 = One Button Dialog(message=w285) -> ()  [unwired: 2 out]
              }
              frame #1 {
              }
            }
            "Flight Software Version" <- w282
          }
          frame #1 {
            n169 = Increment(x=w292) -> (x+1=w288:i32)
            n170 = Less?(x=w292, y=w298) -> (x < y?=w296:bool)
            n171 = Format Into String(format string="Status:Connection Attempt #%d ...", w288) -> (resulting string=w290:string)  [unwired: 2 in, 1 out]
            n172 = Build Array(w290, "Connect to AeroQuad") -> (w289:string[])
            n173 = Select(t=w289, s=w296, f=string[] ["Disconnect", "Status:Not Connected to AeroQuad", "Connection Retry Dialog:Startup"]) -> (s? t:f=w294:string[])
            n174 = Increment(x=w292) -> (x+1=w297:i32)
          }
        }
        n175 = for {
          tunnel: w278 -> [w300] mode=indexing
          tunnel: w277 -> [w299]
          n176 = Enqueue Element(queue=w299, element=w300) -> ()  [unwired: 1 in, 4 out]
        }
        n177 = Bundle By Name(cluster=w262, "CurrentRetry"=w259, "Error"=w260) -> (w256:T11)
      }
      frame #17 {
        n178 = Unbundle By Name(w304) -> ("Connected"=w303:bool, "COMport"=w302:refnum<visa-resource-name>, "Timeout"=w301:u32)
        n179 = case shown="True" w303 {
          tunnel: [w306 w321] -> w305
          tunnel: w304 -> [w306 w320]
          tunnel: w302 -> [_ w310]
          tunnel: w301 -> [_ w308]
          frame #0 {
          }
          frame #1 {
            n180 = property class="Instr"(reference=w310, "Timeout"=w308) -> (reference out=w309:refnum<visa-resource-name>, error out=w307:errorcluster)  [unwired: 1 in]
            n181 = VISA Write(VISA resource name=w309, write buffer="X", error in (no error)=w307) -> (VISA resource name out=w316:refnum<visa-resource-name>, error out=w318:errorcluster)  [unwired: 1 out]
            n182 = call "Time Delay"("error in (no error)"=w318) -> ("error out"=w317:errorcluster)  [unwired: 1 in, 9 out]
            n183 = VISA Flush I/O Buffer(VISA resource name=w316, error in (no error)=w317) -> (VISA resource name out=w314:refnum<visa-resource-name>, error out=w315:errorcluster)  [unwired: 1 in]
            n184 = for {
              shift-right: [w329] -> w311
              shift-left: w315 -> [w333]
              tunnel: w314 -> [w332]
              tunnel: [w330] -> _
              tunnel: string[] ["B", "D", "J", "L", "F", "H", "N"] -> [w328] mode=indexing
              i -> [w323]
              n185 = VISA Write(VISA resource name=w332, write buffer=w328, error in (no error)=w333) -> (VISA resource name out=w334:refnum<visa-resource-name>, error out=w335:errorcluster)  [unwired: 1 out]
              n186 = VISA Read(VISA resource name=w334, byte count=u32 1024, error in (no error)=w335) -> (VISA resource name out=w330:refnum<visa-resource-name>, read buffer=w324:string, error out=w331:errorcluster)  [unwired: 1 out]
              n187 = Spreadsheet String To Array(delimiter (Tab)=",", format string="%.2f", spreadsheet string=w324, array type (2D Dbl)=dbl[] []) -> (array=w322:dbl[])
              n188 = call "Time Delay6"("error in (no error)"=w331) -> ("error out"=w329:errorcluster)  [unwired: 1 in, 9 out]
              n189 = case shown="0, Default" w323 {
                tunnel: w322 -> [w343 w350 w353 w356 w358 w365 w374]
                frame #0 {
                  n190 = Index Array(array=w343) -> (element #1=w342:dbl, element #2=w341:dbl, element #3=w340:dbl, element #4=w339:dbl, element #5=w338:dbl, element #6=w337:dbl)  [unwired: 6 in]
                  n191 = local write "Proportional Roll"(w342) -> ()
                  n192 = local write "Integral Roll"(w341) -> ()
                  n193 = local write "Derivative Roll"(w340) -> ()
                  n194 = local write "ProportionalPitch"(w339) -> ()
                  n195 = local write "IntegralPitch"(w338) -> ()
                  n196 = local write "DerivativePitch"(w337) -> ()
                }
                frame #1 {
                  n197 = Index Array(array=w350) -> (element #1=w348:dbl, element #2=w349:dbl, element #3=w347:dbl, element #4=w346:dbl, element #5=w345:dbl, element #6=w344:dbl)  [unwired: 6 in]
                  n198 = local write "ProportionalHeading"(w346) -> ()
                  n199 = local write "IntegralHeading"(w345) -> ()
                  n200 = local write "DerivativeHeading"(w344) -> ()
                  n201 = local write "ProportionalYaw"(w348) -> ()
                  n202 = local write "IntegralYaw"(w349) -> ()
                  n203 = local write "DerivativeYaw"(w347) -> ()
                }
                frame #2 {
                  n204 = Index Array(array=w353) -> (element #1=w352:dbl, element #2=w351:dbl)  [unwired: 2 in]
                  n205 = local write "Windup Guard"(w352) -> ()
                  n206 = local write "Transmitter Factor"(w351) -> ()
                }
                frame #3 {
                  n207 = Index Array(array=w356) -> (element #1=w354:dbl, element #2=w357:dbl, element #3=w355:dbl)  [unwired: 3 in]
                  n208 = local write "Gyro Smooth Factor"(w354) -> ()
                  n209 = local write "Acc Smooth Factor"(w357) -> ()
                  n210 = local write "Complementary Filter"(w355) -> ()
                }
                frame #4 {
                  n211 = Index Array(array=w358) -> (element #1=w364:dbl, element #2=w363:dbl, element #3=w362:dbl, element #4=w361:dbl, element #5=w360:dbl, element #6=w359:dbl)  [unwired: 6 in]
                  n212 = local write "ProportionalRollLevel"(w364) -> ()
                  n213 = local write "IntegralRollLevel"(w363) -> ()
                  n214 = local write "DerivativeRollLevel"(w362) -> ()
                  n215 = local write "ProportionalPitchLevel"(w361) -> ()
                  n216 = local write "IntegralPitchLevel"(w360) -> ()